vi "FlexMag - 24-03-2023.vi"() -> ()   [LabVIEW 2018] (continued)
                n19188 = flat-sequence {
                  frame #0 {
                    w23535 = sgl 0.5 ("TC2_overspeed_value")
                    n19189 = local read "tension value"() -> (w23537:dbl)
                    n19190 = Wait (ms)(milliseconds to wait=u32 300) -> ()  [unwired: 1 out]
                    n19191 = local write "TC1_set_value"(w23537) -> ()
                    n19192 = local write "TC2_overspeed_value"(w23535) -> ()
                    n19193 = local write "current voltage"(w23535) -> ()
                  }
                  frame #1 {
                    n19194 = local write "TC2_overspeed_set"(TRUE ("TC2 Set moxa")) -> ()
                    n19195 = local write "TC1_auto_set"(TRUE ("TC1_set")) -> ()
                  }
                  frame #2 {
                    n19196 = local write "TC1_overspeed_value"(sgl 0.0 ("TC2_set_value")) -> ()
                    n19197 = local write "TC2_set_value"(sgl 0.0 ("TC2_set_value")) -> ()
                    n19198 = Wait (ms)(milliseconds to wait=u32 300) -> ()  [unwired: 1 out]
                  }
                  frame #3 {
                    n19199 = local write "TC2_auto_set"(TRUE ("TC2_auto_set")) -> ()
                    n19200 = local write "TC1_overspeed_set"(TRUE ("TC2_auto_set")) -> ()
                  }
                }
              }
            }
          }
          frame #10 {
            n19201 = local read "position"() -> (w23545:bool)
            n19202 = case shown="True" w23545 {
              frame False {
              }
              frame True {
                w23547 = TRUE ("CH1_SRV_Direction_Clockwise_DO")
                n19203 = local write "CH1_SRV_Direction_Clockwise_DO"(w23547) -> ()
                n19204 = local write "CH2_SRV_Direction_Clockwise_DO"(w23547) -> ()
                n19205 = local write "CH3_SRV_Direction_Clockwise_DO"(w23547) -> ()
                n19206 = local write "CH4_SRV_Direction_Clockwise_DO"(w23547) -> ()
                n19207 = Wait (ms)(milliseconds to wait=u32 100) -> ()  [unwired: 1 out]
              }
            }
          }
          frame #11 {
            n19208 = local read "position"() -> (w23548:bool)
            n19209 = case shown="True" w23548 {
              frame False {
              }
              frame True {
                n19210 = local write "Tension_Controllers_Start/Stop DO"(TRUE ("CH1_SRV_Direction_Clockwise_DO")) -> ()
                n19211 = Wait (ms)(milliseconds to wait=u32 100) -> ()  [unwired: 1 out]
              }
            }
          }
          frame #12 {
            n19212 = local read "position"() -> (w23552:bool)
            n19213 = case shown="True" w23552 {
              tunnel: w23551 -> [_ w23553]
              frame False {
              }
              frame True {
                n19214 = Wait (ms)(milliseconds to wait=u32 100) -> ()  [unwired: 1 out]
                n19215 = case shown="0, Default" w23553 {
                  frame 0, Default {
                    n19216 = local write "roll error"(TRUE ("roll error")) -> ()
                  }
                  frame 1 {
                    n19217 = local write "CH1_Motor DO"(TRUE ("CH1_Motor DO")) -> ()
                  }
                  frame 2 {
                    n19218 = local write "CH2_Motor DO"(TRUE ("CH1_Motor DO")) -> ()
                  }
                  frame 3 {
                    n19219 = local write "CH3_Motor DO"(TRUE ("CH1_Motor DO")) -> ()
                  }
                  frame 4 {
                    n19220 = local write "CH4_Motor DO"(TRUE ("CH1_Motor DO")) -> ()
                  }
                }
              }
            }
          }
          frame #13 {
            n19221 = stacked-sequence {
              tunnel: w23560 -> [w23561 w23596 _]
              frame #0 {
                n19222 = local read "position"() -> (w23562:bool)
                n19223 = case shown="True" w23562 {
                  tunnel: w23561 -> [_ w23563]
                  frame False {
                  }
                  frame True {
                    n19224 = case shown="4" w23563 {
                      frame 0, Default {
                      }
                      frame 1 {
                        n19225 = while {
                          stop <- w23566 stop-if-true
                          n19226 = local read "Ch1_srv1_counter DI"() -> (w23569:bool)
                          n19227 = Wait Until Next ms Multiple(millisecond multiple=u32 100) -> ()  [unwired: 1 out]
                          n19228 = local read "position"() -> (w23567:bool)
                          n19229 = case shown="True" w23569 {
                            tunnel: [FALSE TRUE] -> w23565
                            frame False {
                            }
                            frame True {
                            }
                          }
                          n19230 = Not(x=w23567) -> (.not. x?=w23564:bool)
                          n19231 = Or(x=w23565, y=w23564) -> (x .or. y?=w23566:bool)
                        }
                      }
                      frame 2 {
                        n19232 = while {
                          stop <- w23574 stop-if-true
                          n19233 = local read "Ch2_srv1_counter DI"() -> (w23577:bool)
                          n19234 = Wait Until Next ms Multiple(millisecond multiple=u32 100) -> ()  [unwired: 1 out]
                          n19235 = local read "position"() -> (w23575:bool)
                          n19236 = case shown="True" w23577 {
                            tunnel: [FALSE TRUE] -> w23573
                            frame False {
                            }
                            frame True {
                            }
                          }
                          n19237 = Not(x=w23575) -> (.not. x?=w23572:bool)
                          n19238 = Or(x=w23573, y=w23572) -> (x .or. y?=w23574:bool)
                        }
                      }
                      frame 3 {
                        n19239 = while {
                          stop <- w23582 stop-if-true
                          n19240 = local read "Ch3_srv1_counter DI"() -> (w23585:bool)
                          n19241 = Wait Until Next ms Multiple(millisecond multiple=u32 100) -> ()  [unwired: 1 out]
                          n19242 = local read "position"() -> (w23583:bool)
                          n19243 = case shown="True" w23585 {
                            tunnel: [FALSE TRUE] -> w23581
                            frame False {
                            }
                            frame True {
                            }
                          }
                          n19244 = Not(x=w23583) -> (.not. x?=w23580:bool)
                          n19245 = Or(x=w23581, y=w23580) -> (x .or. y?=w23582:bool)
                        }
                      }
                      frame 4 {
                        n19246 = while {
                          stop <- w23590 stop-if-true
                          n19247 = local read "Ch4_srv1_counter DI"() -> (w23593:bool)
                          n19248 = Wait Until Next ms Multiple(millisecond multiple=u32 100) -> ()  [unwired: 1 out]
                          n19249 = local read "position"() -> (w23591:bool)
                          n19250 = case shown="True" w23593 {
                            tunnel: [FALSE TRUE] -> w23589
                            frame False {
                            }
                            frame True {
                            }
                          }
                          n19251 = Not(x=w23591) -> (.not. x?=w23588:bool)
                          n19252 = Or(x=w23589, y=w23588) -> (x .or. y?=w23590:bool)
                        }
                      }
                    }
                  }
                }
              }
              frame #1 {
                n19253 = local read "position"() -> (w23597:bool)
                n19254 = case shown="True" w23597 {
                  tunnel: w23596 -> [_ w23598]
                  frame False {
                  }
                  frame True {
                    n19255 = case shown="0, Default" w23598 {
                      frame 0, Default {
                        n19256 = local write "roll error"(TRUE ("roll error")) -> ()
                      }
                      frame 1 {
                        n19257 = while {
                          stop <- w23602 stop-if-true
                          n19258 = local read "Ch1_srv1_counter DI"() -> (w23605:bool)
                          n19259 = Wait Until Next ms Multiple(millisecond multiple=u32 100) -> ()  [unwired: 1 out]
                          n19260 = local read "position"() -> (w23603:bool)
                          n19261 = case shown="False" w23605 {
                            tunnel: [TRUE FALSE] -> w23601
                            frame False {
                              n19262 = local write "CH1_Motor DO"(FALSE ("CH1_Motor DO")) -> ()
                            }
                            frame True {
                            }
                          }
                          n19263 = Not(x=w23603) -> (.not. x?=w23600:bool)
                          n19264 = Or(x=w23601, y=w23600) -> (x .or. y?=w23602:bool)
                        }
                      }
                      frame 2 {
                        n19265 = while {
                          stop <- w23611 stop-if-true
                          n19266 = local read "Ch2_srv1_counter DI"() -> (w23614:bool)
                          n19267 = Wait Until Next ms Multiple(millisecond multiple=u32 100) -> ()  [unwired: 1 out]
                          n19268 = local read "position"() -> (w23612:bool)
                          n19269 = case shown="False" w23614 {
                            tunnel: [TRUE FALSE] -> w23610
                            frame False {
                              n19270 = local write "CH2_Motor DO"(FALSE ("CH1_Motor DO")) -> ()
                            }
                            frame True {
                            }
                          }
                          n19271 = Not(x=w23612) -> (.not. x?=w23609:bool)
                          n19272 = Or(x=w23610, y=w23609) -> (x .or. y?=w23611:bool)
                        }
                      }
                      frame 3 {
                        n19273 = while {
                          stop <- w23620 stop-if-true
                          n19274 = local read "Ch3_srv1_counter DI"() -> (w23623:bool)
                          n19275 = Wait Until Next ms Multiple(millisecond multiple=u32 100) -> ()  [unwired: 1 out]
                          n19276 = local read "position"() -> (w23621:bool)
                          n19277 = case shown="False" w23623 {
                            tunnel: [TRUE FALSE] -> w23619
                            frame False {
                              n19278 = local write "CH3_Motor DO"(FALSE ("CH1_Motor DO")) -> ()
                            }
                            frame True {
                            }
                          }
                          n19279 = Not(x=w23621) -> (.not. x?=w23618:bool)
                          n19280 = Or(x=w23619, y=w23618) -> (x .or. y?=w23620:bool)
                        }
                      }
                      frame 4 {
                        n19281 = while {
                          stop <- w23629 stop-if-true
                          n19282 = local read "Ch4_srv1_counter DI"() -> (w23632:bool)
                          n19283 = Wait Until Next ms Multiple(millisecond multiple=u32 100) -> ()  [unwired: 1 out]
                          n19284 = local read "position"() -> (w23630:bool)
                          n19285 = case shown="False" w23632 {
                            tunnel: [TRUE FALSE] -> w23628
                            frame False {
                              n19286 = local write "CH4_Motor DO"(FALSE ("CH1_Motor DO")) -> ()
                            }
                            frame True {
                            }
                          }
                          n19287 = Not(x=w23630) -> (.not. x?=w23627:bool)
                          n19288 = Or(x=w23628, y=w23627) -> (x .or. y?=w23629:bool)
                        }
                      }
                    }
                  }
                }
              }
              frame #2 {
                w23636 = FALSE ("forward roll")
                n19289 = local write "Tension_Controllers_Start/Stop DO"(w23636) -> ()
                n19290 = local write "CH1_Motor DO"(w23636) -> ()
                n19291 = local write "CH2_Motor DO"(w23636) -> ()
                n19292 = local write "CH3_Motor DO"(w23636) -> ()
                n19293 = local write "CH4_Motor DO"(w23636) -> ()
                n19294 = local write "position"(FALSE ("position")) -> ()
                n19295 = Wait (ms)(milliseconds to wait=u32 300) -> ()  [unwired: 1 out]
              }
            }
          }
        }
      }
    }
  }
  n19296 = while {
    stop <- FALSE stop-if-true
    n19297 = Wait Until Next ms Multiple(millisecond multiple=u32 300) -> ()  [unwired: 1 out]
    n19298 = case shown="True" "calculate" {
      frame False {
      }
      frame True {
        n19299 = stacked-sequence {
          frame #0 {
            w23643 = 0.0 ("lap number right target")
            n19300 = local read "initial right diameter"() -> (w23642:dbl)
            n19301 = local write "final right diameter"(w23642) -> ()
            n19302 = local write "lap number right target"(w23643) -> ()
            n19303 = local write "total interval"(w23643) -> ()
          }
          frame #1 {
            n19304 = while {
              stop <- w23654 stop-if-true
              n19305 = local read "web thickness"() -> (w23651:dbl)
              n19306 = local read "final right diameter"() -> (w23645:dbl)
              n19307 = local read "lap number right target"() -> (w23659:dbl)
              n19308 = local read "total interval"() -> (w23648:dbl)
              n19309 = Multiply(x=w23651, y=0.002) -> (x*y=w23652:dbl)
              n19310 = Multiply(x=w23645, y=0.1) -> (x*y=w23646:dbl)
              n19311 = local read "target interval"() -> (w23655:dbl)
              n19312 = Add(x=w23645, y=w23652) -> (x+y=w23653:dbl)
              n19313 = Multiply(x=3.141592653589793, y=w23646) -> (x*y=w23649:dbl)
              n19314 = Add(x=w23659, y=1.0) -> (x+y=w23660:dbl)
              n19315 = local write "lap number right target"(w23660) -> ()
              n19316 = local write "final right diameter"(w23653) -> ()
              n19317 = Add(x=w23648, y=w23649) -> (x+y=w23647:dbl)
              n19318 = Greater Or Equal?(x=w23647, y=w23655) -> (x >= y?=w23654:bool)
              n19319 = local write "total interval"(w23647) -> ()
              n19320 = Wait Until Next ms Multiple(millisecond multiple=u32 50) -> ()  [unwired: 1 out]
            }
          }
          frame #2 {
            n19321 = local read "initial right diameter"() -> (w23673:dbl)
            n19322 = local read "final right diameter"() -> (w23661:dbl)
            n19323 = local read "web speed"() -> (w23670:dbl)
            n19324 = local read "web speed"() -> (w23662:dbl)
            n19325 = Multiply(x=w23673, y=3.141592653589793) -> (x*y=w23671:dbl)
            n19326 = Multiply(x=w23661, y=3.141592653589793) -> (x*y=w23674:dbl)
            n19327 = Divide(x=w23670, y=w23671) -> (x/y=w23667:dbl)
            n19328 = Divide(x=w23662, y=w23674) -> (x/y=w23669:dbl)
            n19329 = Multiply(x=w23669, y=10.0) -> (x*y=→"min circular speed":dbl)
            n19330 = Multiply(x=w23667, y=10.0) -> (x*y=→"max circular speed":dbl)
            n19331 = Wait (ms)(milliseconds to wait=u32 100) -> ()  [unwired: 1 out]
          }
          frame #3 {
            # "1/50 redüktör"
            # "1000rpm 10volts"
            n19332 = local read "min circular speed"() -> (w23681:dbl)
            n19333 = local read "max circular speed"() -> (w23685:dbl)
            n19334 = Multiply(x=0.01, y=50.0 ("x")) -> (x*y=w23682:dbl)
            n19335 = Multiply(x=w23685, y=w23682) -> (x*y=w23676:dbl)
            n19336 = Multiply(x=w23682, y=w23681) -> (x*y=w23677:dbl)
            n19337 = local write "final output voltage"(w23677) -> ()
            n19338 = local read "lap number right target"() -> (w23679:dbl)
            n19339 = Subtract(x=w23676, y=w23677) -> (x-y=w23680:dbl)
            n19340 = local write "initial output voltage"(w23676) -> ()
            n19341 = Divide(x=w23680, y=w23679) -> (x/y=w23678:dbl)
            n19342 = local write "decreasing voltage"(w23678) -> ()
          }
          frame #4 {
            n19343 = local write "calculate"(FALSE ("calculate")) -> ()
          }
        }
      }
    }
  }
  n19344 = while {
    stop <- FALSE stop-if-true
    n19345 = Wait Until Next ms Multiple(millisecond multiple=u32 300) -> ()  [unwired: 1 out]
    n19346 = case shown="True" "tension check active" {
      frame False {
      }
      frame True {
        n19347 = local read "Tension_Controllers_Start/Stop DO"() -> (w23718:bool)
        n19348 = local read "CH1_Motor DO"() -> (w23723:bool)
        n19349 = local read "CH2_Motor DO"() -> (w23722:bool)
        n19350 = local read "CH3_Motor DO"() -> (w23721:bool)
        n19351 = local read "CH4_Motor DO"() -> (w23720:bool)
        n19352 = Compound Arithmetic op=OR(w23723, w23722, w23721, w23720) -> (w23717:bool)
        n19353 = And(x=w23718, y=w23717) -> (x .and. y?=w23719:bool)
        n19354 = feedback #338() -> (w23715:bool)  [unwired: 1 in]
        n19355 = case shown="True" w23719 {
          tunnel: [TRUE ("Dc_auto_off") w23729] -> w23716
          tunnel: w23715 -> [_ w23728]
          tunnel: "check both tensions" -> [_ w23727]
          frame False {
          }
          frame True {
            n19356 = case shown="True" w23727 {
              tunnel: "tension check value" -> [w23731 w23739]
              tunnel: [w23730 w23736] -> w23725
              frame False {
                n19357 = local read "forward roll"() -> (w23733:bool)
                n19358 = case shown="False" w23733 {
                  tunnel: [w23734 w23735] -> w23732
                  frame False {
                    n19359 = local read "TC2_measure_value"() -> (w23734:sgl)
                  }
                  frame True {
                    n19360 = local read "TC1_measure_value"() -> (w23735:sgl)
                  }
                }
                n19361 = Greater Or Equal?(x=w23732, y=w23731) -> (x >= y?=w23730:bool)
              }
              frame True {
                n19362 = local read "TC1_measure_value"() -> (w23741:sgl)
                n19363 = local read "TC2_measure_value"() -> (w23740:sgl)
                n19364 = Greater Or Equal?(x=w23741, y=w23739) -> (x >= y?=w23738:bool)
                n19365 = Greater Or Equal?(x=w23740, y=w23739) -> (x >= y?=w23737:bool)
                n19366 = Or(x=w23738, y=w23737) -> (x .or. y?=w23736:bool)
              }
            }
            n19367 = case shown="True" w23725 {
              tunnel: [TRUE ("Dc_auto_off") FALSE] -> w23729
              tunnel: w23728 -> [_ w23743]
              frame False {
              }
              frame True {
                n19368 = call "Elapsed Time191"("Reset"=w23743) -> ("Elapsed Time (s)"=w23746:dbl)  [unwired: 11 in, 7 out]
                n19369 = Greater?(x=w23746, y="tension check (sec)") -> (0:w23744:bool)
                n19370 = case shown="True" w23744 {
                  frame False {
                  }
                  frame True {
                    n19371 = local write "Warning Message"("Rolling Problem !\nToo much Tension !" ("Warning Message")) -> ()
                    n19372 = local write "roll error"(TRUE ("roll error")) -> ()
                  }
                }
              }
            }
          }
        }
        n19373 = feedback-in #338(w23716) -> ()
      }
    }
    n19374 = case shown="True" "speed check active" {
      frame False {
      }
      frame True {
        n19375 = local read "Tension_Controllers_Start/Stop DO"() -> (w23698:bool)
        n19376 = local read "CH1_Motor DO"() -> (w23694:bool)
        n19377 = local read "CH2_Motor DO"() -> (w23695:bool)
        n19378 = local read "CH3_Motor DO"() -> (w23696:bool)
        n19379 = local read "CH4_Motor DO"() -> (w23697:bool)
        n19380 = Compound Arithmetic op=OR(w23694, w23695, w23696, w23697) -> (w23699:bool)
        n19381 = feedback #339() -> (w23691:bool)  [unwired: 1 in]
        n19382 = And(x=w23698, y=w23699) -> (x .and. y?=w23693:bool)
        n19383 = case shown="True" w23693 {
          tunnel: [TRUE ("Dc_auto_off") w23702] -> w23692
          tunnel: w23691 -> [_ w23701]
          frame False {
          }
          frame True {
            n19384 = local read "process variable"() -> (w23705:dbl)
            n19385 = Less Or Equal?(x=w23705, y="speed compare value") -> (x <= y?=w23703:bool)
            n19386 = case shown="True" w23703 {
              tunnel: [TRUE ("Dc_auto_off") FALSE] -> w23702
              tunnel: w23701 -> [_ w23710]
              frame False {
              }
              frame True {
                n19387 = call "Elapsed Time193"("Reset"=w23710) -> ("Elapsed Time (s)"=w23709:dbl)  [unwired: 11 in, 7 out]
                n19388 = Greater?(x=w23709, y="speed check (sec)") -> (0:w23707:bool)
                n19389 = case shown="True" w23707 {
                  frame False {
                  }
                  frame True {
                    n19390 = local write "roll error"(TRUE ("roll error")) -> ()
                    n19391 = local write "Warning Message"("Rolling Problem !\nNo Speed !" ("Warning Message")) -> ()
                  }
                }
              }
            }
          }
        }
        n19392 = feedback-in #339(w23692) -> ()
      }
    }
  }
  n19393 = while {
    stop <- FALSE stop-if-true
    n19394 = flat-sequence {
      frame #0 {
        n19395 = local read "keysight readout"() -> (w23760:dbl)
        n19396 = In Range and Coerce(upper limit="output limit max", x=w23760, lower limit="output limit min") -> (coerced(x)=w23754:dbl)  [unwired: 1 out]
        "freq readout" <- w23754
        n19397 = Divide(x="speed coef", y="freq coef") -> (x/y=w23755:sgl)
        n19398 = Multiply(x=w23754, y=w23755) -> (x*y=→"process variable":dbl)
      }
      frame #1 {
        n19399 = local read "process variable"() -> (w23761:dbl)
        n19400 = call-poly <vilib>:"PID.vi"("output range"="output range", "dt (s)"="dt (s)", "PID gains"="PID gains", "process variable"=w23761, "setpoint"="setpoint") -> ("output"=→"output_pid" →"Waveform Chart":dbl)  [unwired: 5 in, 1 out]
      }
    }
    n19401 = Wait Until Next ms Multiple(millisecond multiple=u32 300) -> ()  [unwired: 1 out]
    n19402 = property on="pid graph" class="TabCtl (strict)"("Visible"="show graph") -> ()  [unwired: 2 in, 2 out]
  }
  n19403 = disable-structure shown="Disabled" {
    frame Disabled {
      n19404 = while {
        stop <- FALSE stop-if-true
        n19405 = Wait Until Next ms Multiple(millisecond multiple=u32 300) -> ()  [unwired: 1 out]
        n19406 = case shown="True" "pid output" {
          frame False {
          }
          frame True {
            n19407 = stacked-sequence {
              frame #0 {
                n19408 = while {
                  i -> [w23776]
                  stop <- w23771 stop-if-true
                  n19409 = local read "final output voltage"() -> (w23773:dbl)
                  n19410 = Wait Until Next ms Multiple(millisecond multiple=u32 300) -> ()  [unwired: 1 out]
                  n19411 = Multiply(x=w23776, y=0.5 ("lower limit")) -> (x*y=w23774:dbl)
                  n19412 = Greater Or Equal?(x=w23774, y=w23773) -> (x >= y?=w23772:bool)
                  n19413 = In Range and Coerce(upper limit=w23773, x=w23774, lower limit=0.5) -> (coerced(x)=w23770:dbl)  [unwired: 1 out]
                  n19414 = case shown="True" w23772 {
                    tunnel: [FALSE ("pid output") TRUE ("pid output")] -> w23771
                    frame False {
                    }
                    frame True {
                      n19415 = local write "pid output"(FALSE ("pid output")) -> ()
                    }
                  }
                  n19416 = Bundle("final output voltage"=w23770, "final output voltage"=w23770) -> (w23779:T17)  [unwired: 1 in]
                  n19417 = local write "output range"(w23779) -> ()
                }
              }
              frame #1 {
                n19418 = local read "initial output voltage"() -> (w23785:dbl)
                n19419 = local read "final output voltage"() -> (w23784:dbl)
                n19420 = Wait (ms)(milliseconds to wait=u32 100) -> ()  [unwired: 1 out]
                n19421 = Bundle("initial output voltage"=w23785, "final output voltage"=w23784) -> (w23786:T18)  [unwired: 1 in]
                n19422 = local write "output range"(w23786) -> ()
              }
            }
          }
        }
      }
    }
    frame Enabled {
    }
  }
  n19423 = local write "dep. for?"(w1) -> ()
  n19424 = while {
    stop <- FALSE stop-if-true
    n19425 = local read "process file list"() -> (w23790:string)
    n19426 = Wait Until Next ms Multiple(millisecond multiple=u32 300) -> ()  [unwired: 1 out]
    n19427 = Match Pattern(string=w23790, regular expression="\r\n") -> (before substring=w23791:string)  [unwired: 1 in, 3 out]
    n19428 = Equal?(x=w23791, y="FlexMag Process File") -> (x = y?=w23787:bool)
    n19429 = case shown="True" "coating start" {
      tunnel: w23787 -> [_ w23796]
      frame False {
      }
      frame True {
        n19430 = case shown="True" w23796 {
          frame False {
            n19431 = flat-sequence {
              frame #0 {
                n19432 = local write "Buzzer DO"(TRUE ("Buzzer DO")) -> ()
                n19433 = local write "coating start"(FALSE ("coating start")) -> ()
                n19434 = local write "Warning Message"("Please Enter a proper Process File !" ("Warning Message")) -> ()
              }
              frame #1 {
                n19435 = Wait (ms)(milliseconds to wait=u32 3000) -> ()  [unwired: 1 out]
              }
              frame #2 {
                n19436 = local write "Buzzer DO"(FALSE ("Buzzer DO")) -> ()
              }
            }
          }
          frame True {
            n19437 = while {
              i -> [w23809]
              stop <- "coating process done" stop-if-true
              n19438 = Increment(x=w23809) -> (x+1=w23804:i32)
              n19439 = local read "process file list"() -> (w23817:string)
              n19440 = Number To Decimal String(number=w23804) -> (decimal integer string=w23816:string)  [unwired: 1 in]
              n19441 = Concatenate Strings(w23816, "-)") -> (w23814:string)
              n19442 = Wait Until Next ms Multiple(millisecond multiple=u32 300) -> ()  [unwired: 1 out]
              n19443 = Increment(x=w23804) -> (x+1=w23807:i32)
              n19444 = Match Pattern(string=w23817, regular expression=w23814) -> (after substring=w23813:string)  [unwired: 1 in, 3 out]
              n19445 = Number To Decimal String(number=w23807) -> (decimal integer string=w23806:string)  [unwired: 1 in]
              n19446 = Concatenate Strings(w23806, "-)") -> (w23803:string)
              n19447 = Match Pattern(string=w23813, regular expression=w23803) -> (before substring=w23808:string)  [unwired: 1 in, 3 out]
              n19448 = Equal?(x="", y=w23808) -> (x = y?=w23811:bool)
              n19449 = case shown="False" w23811 {
                tunnel: w23808 -> [w23819 _]
                tunnel: w23804 -> [w23818 _]
                frame False {
                  # "process available"
                  n19450 = stacked-sequence {
                    tunnel: w23819 -> [w23825 _]
                    tunnel: w23818 -> [w23821 _]
                    frame #0 {
                      n19451 = local read "coating start"() -> (w23820:bool)
                      n19452 = case shown="False" w23820 {
                        tunnel: [w23828 w23829] -> w23822
                        tunnel: w23821 -> [_ w23829]
                        frame False {
                          n19453 = local read "current recipe number"() -> (w23828:i32)
                        }
                        frame True {
                        }
                      }
                      "current recipe number" <- w23822
                      n19454 = local read "cassette position selection"() -> (w23823:u16)
                      n19455 = Match Pattern(string=w23825, regular expression="\r\n") -> (before substring=w23826:string)  [unwired: 1 in, 3 out]
                      "process file list 2" <- w23826
                      n19456 = case shown="0, Default" w23823 {
                        frame 0, Default {
                          n19457 = local write "coating error"(TRUE ("coating error")) -> ()
                          n19458 = local write "Warning Message"("Choose Cassette Position !" ("Warning Message")) -> ()
                        }
                        frame 1 {
                        }
                        frame 2 {
                        }
                        frame 3 {
                        }
                        frame 4 {
                        }
                      }
                      n19459 = stacked-sequence {
                        tunnel: w23826 -> [w23834 _ _ _ _]
                        frame #0 {
                          n19460 = String To Path(string=w23834) -> (path=→"path for loading recipe":path)
                          n19461 = Wait (ms)(milliseconds to wait=u32 500) -> ()  [unwired: 1 out]
                        }
                        frame #1 {
                          n19462 = Wait (ms)(milliseconds to wait=u32 1000) -> ()  [unwired: 1 out]
                        }
                        frame #2 {
                          n19463 = local write "load recipe from path"(TRUE ("load recipe from path")) -> ()
                        }
                        frame #3 {
                          n19464 = Wait (ms)(milliseconds to wait=u32 1000) -> ()  [unwired: 1 out]
                        }
                        frame #4 {
                          n19465 = while {
                            i -> [w23840]
                            stop <- w23844 stop-if-true
                            n19466 = local read "load recipe from path"() -> (w23841:bool)
                            n19467 = local read "ABORT"() -> (w23843:bool)
                            n19468 = Wait Until Next ms Multiple(millisecond multiple=u32 1000) -> ()  [unwired: 1 out]
                            n19469 = Greater?(x=w23840, y=u32 30 ("millisecond multiple")) -> (0:w23838:bool)
                            n19470 = Not(x=w23841) -> (.not. x?=w23842:bool)
                            n19471 = Compound Arithmetic op=OR(w23842, w23843, w23838) -> (w23844:bool)
                            n19472 = local write "coating error"(w23838) -> ()
                          }
                        }
                      }
                      n19473 = local write "System Status"("COATING MODE ACTIVE" ("System Status")) -> ()
                    }
                    frame #1 {
                      n19474 = local read "R Recipe Selection"() -> (w23846:u16)
                      n19475 = case shown="0, Default" w23846 {
                        frame 0, Default {
                          # "SINGLE PROCESS"
                          n19476 = local read "R single process selection"() -> (w23847:enum32{"microwave", "dcsputter", "rfsputter"})
                          n19477 = case shown="\"dcsputter\"" w23847 {
                            frame "microwave", Default {
                            }
                            frame "dcsputter" {
                              # "DC SPUTTER"
                              n19478 = local read "R DC Sputter Chamber Selection"() -> (w23848:enum32{"chamber II", "chamber III"})
                              n19479 = case shown="\"chamber III\"" w23848 {
                                frame "chamber II", Default {
                                # "CH II"
                                n19480 = disable-structure shown="Enabled" {
                                disable-tunnel: [w23850 TRUE] -> w23849
                                frame Disabled {
                                n19481 = local read "ch2 ch pg torr"() -> (w23852:dbl)
                                n19482 = local read "ch2 cc torr"() -> (w23851:dbl)
                                n19483 = Less Or Equal?(x=w23852, y=0.005) -> (x <= y?=w23855:bool)
                                n19484 = Less Or Equal?(x=w23851, y=0.005) -> (x <= y?=w23856:bool)
                                n19485 = And(x=w23855, y=w23856) -> (x .and. y?=w23850:bool)
                                }
                                frame Enabled {
                                }
                                }
                                n19486 = case shown="True" w23849 {
                                frame False {
                                n19487 = local write "coating error"(TRUE ("coating error")) -> ()
                                n19488 = local write "Warning Message"("Automatic Coating Process is canceled !\nCH2 Pressure should be under 5E-3 Torr .." ("Warning Message")) -> ()
                                }
                                frame True {
                                n19489 = stacked-sequence {
                                frame #0 {
                                }
                                frame #1 {
                                n19490 = stacked-sequence {
                                frame #0 {
                                n19491 = local read "abort ch2"() -> (w23860:bool)
                                n19492 = case shown="False" w23860 {
                                frame False {
                                n19493 = local read "coating start"() -> (w23861:bool)
                                n19494 = case shown="True" w23861 {
                                frame False {
                                }
                                frame True {
                                n19495 = local read "casette_ch2_gui"() -> (w23863:bool)
                                n19496 = Wait (ms)(milliseconds to wait=u32 100) -> ()  [unwired: 1 out]
                                n19497 = case shown="False" w23863 {
                                frame False {
                                n19498 = stacked-sequence {
                                frame #0 {
                                n19499 = flat-sequence {
                                frame #0 {
                                n19500 = local write "target chamber"(2.0 ("target chamber")) -> ()
                                n19501 = Wait (ms)(milliseconds to wait=u32 100) -> ()  [unwired: 1 out]
                                }
                                frame #1 {
                                n19502 = Wait (ms)(milliseconds to wait=u32 1000) -> ()  [unwired: 1 out]
                                }
                                frame #2 {
                                n19503 = local write "transfer vacuum auto"(TRUE ("transfer vacuum")) -> ()
                                }
                                }
                                }
                                frame #1 {
                                n19504 = while {
                                i -> [w23871]
                                stop <- w23873 stop-if-true
                                # "20min"
                                n19505 = local read "present location"() -> (w23877:dbl)
                                n19506 = local read "casette_ch2_gui"() -> (w23869:bool)
                                n19507 = local read "abort ch2"() -> (w23872:bool)
                                n19508 = Equal?(x=w23877, y=2.0) -> (x = y?=w23875:bool)
                                n19509 = Greater?(x=w23871, y=1200) -> (0:w23868:bool)
                                n19510 = local write "trns error"(w23868) -> ()
                                n19511 = Compound Arithmetic op=OR(w23872, w23875, w23869, w23868) -> (w23873:bool)
                                n19512 = Wait Until Next ms Multiple(millisecond multiple=u32 1000) -> ()  [unwired: 1 out]
                                }
                                }
                                }
                                }
                                frame True {
                                }
                                }
                                }
                                }
                                }
                                frame True {
                                }
                                }
                                }
                                frame #1 {
                                n19513 = local read "abort ch2"() -> (w23878:bool)
                                n19514 = case shown="False" w23878 {
                                frame False {
                                n19515 = local read "coating start"() -> (w23879:bool)
                                n19516 = case shown="True" w23879 {
                                frame False {
                                }
                                frame True {
                                n19517 = Wait (ms)(milliseconds to wait=u32 100) -> ()  [unwired: 1 out]
                                n19518 = local write "System Status"("COATING MODE ACTIVE" ("System Status")) -> ()
                                "coating ch2 led 1" <- TRUE ("coating ch2 led 1")
                                }
                                }
                                }
                                frame True {
                                }
                                }
                                }
                                }
                                }
                                frame #2 {
                                # "water"
                                n19519 = stacked-sequence {
                                frame #0 {
                                # "ch1 water off"
                                n19520 = local read "abort ch2"() -> (w23883:bool)
                                n19521 = case shown="False" w23883 {
                                frame False {
                                n19522 = local read "coating start"() -> (w23884:bool)
                                n19523 = case shown="True" w23884 {
                                frame False {
                                }
                                frame True {
                                n19524 = while {
                                i -> [w23887]
                                stop <- w23889 stop-if-true
                                n19525 = Greater Or Equal?(x=w23887, y=100) -> (x >= y?=w23888:bool)
                                n19526 = case shown="True" w23888 {
                                frame False {
                                }
                                frame True {
                                n19527 = local write "coating error"(TRUE ("coating error")) -> ()
                                n19528 = local write "Warning Message"("Automatic Coating Process is canceled !\nCH1 Water Flow Problem.." ("Warning Message")) -> ()
                                }
                                }
                                n19529 = local read "CH1_WFC_DI"() -> (w23893:bool)
                                n19530 = case shown="True" w23893 {
                                tunnel: [TRUE ("CH2_WFC_DO") FALSE ("CH2_WFC_DO")] -> w23892
                                frame False {
                                }
                                frame True {
                                n19531 = Wait Until Next ms Multiple(millisecond multiple=u32 200) -> ()  [unwired: 1 out]
                                n19532 = local write "CH1_WFC_DO"(FALSE ("CH2_WFC_DO")) -> ()
                                }
                                }
                                n19533 = local read "coating start"() -> (w23891:bool)
                                n19534 = local read "abort ch2"() -> (w23885:bool)
                                n19535 = Not(x=w23891) -> (.not. x?=w23890:bool)
                                n19536 = Compound Arithmetic op=OR(w23892, w23890, w23885) -> (w23889:bool)
                                }
                                }
                                }
                                }
                                frame True {
                                }
                                }
                                }
                                frame #1 {
                                # "ch3 water off"
                                n19537 = local read "abort ch2"() -> (w23900:bool)
                                n19538 = case shown="False" w23900 {
                                frame False {
                                n19539 = local read "coating start"() -> (w23901:bool)
                                n19540 = case shown="True" w23901 {
                                frame False {
                                }
                                frame True {
                                n19541 = while {
                                i -> [w23904]
                                stop <- w23906 stop-if-true
                                n19542 = Greater Or Equal?(x=w23904, y=100) -> (x >= y?=w23905:bool)
                                n19543 = case shown="True" w23905 {
                                frame False {
                                }
                                frame True {
                                n19544 = local write "coating error"(TRUE ("coating error")) -> ()
                                n19545 = local write "Warning Message"("Automatic Coating Process is canceled !\nCH3 Water Flow Problem.." ("Warning Message")) -> ()
                                }
                                }
                                n19546 = local read "CH3_WFC_DI"() -> (w23910:bool)
                                n19547 = case shown="True" w23910 {
                                tunnel: [TRUE ("CH2_WFC_DO") FALSE ("CH2_WFC_DO")] -> w23909
                                frame False {
                                }
                                frame True {
                                n19548 = Wait Until Next ms Multiple(millisecond multiple=u32 200) -> ()  [unwired: 1 out]
                                n19549 = local write "CH3_WFC_DO"(FALSE ("CH2_WFC_DO")) -> ()
                                }
                                }
                                n19550 = local read "coating start"() -> (w23908:bool)
                                n19551 = local read "abort ch2"() -> (w23902:bool)
                                n19552 = Not(x=w23908) -> (.not. x?=w23907:bool)
                                n19553 = Compound Arithmetic op=OR(w23909, w23907, w23902) -> (w23906:bool)
                                }
                                }
                                }
                                }
                                frame True {
                                }
                                }
                                }
                                frame #2 {
                                # "ch4 water off"
                                n19554 = local read "abort ch2"() -> (w23917:bool)
                                n19555 = case shown="False" w23917 {
                                frame False {
                                n19556 = local read "coating start"() -> (w23918:bool)
                                n19557 = case shown="True" w23918 {
                                frame False {
                                }
                                frame True {
                                n19558 = while {
                                i -> [w23921]
                                stop <- w23923 stop-if-true
                                n19559 = Greater Or Equal?(x=w23921, y=100) -> (x >= y?=w23922:bool)
                                n19560 = case shown="True" w23922 {
                                frame False {
                                }
                                frame True {
                                n19561 = local write "coating error"(TRUE ("coating error")) -> ()
                                n19562 = local write "Warning Message"("Automatic Coating Process is canceled !\nCH4 Water Flow Problem.." ("Warning Message")) -> ()
                                }
                                }
                                n19563 = local read "CH4_WFC_DI"() -> (w23927:bool)
                                n19564 = case shown="True" w23927 {
                                tunnel: [TRUE ("CH2_WFC_DO") FALSE ("CH2_WFC_DO")] -> w23926
                                frame False {
                                }
                                frame True {
                                n19565 = Wait Until Next ms Multiple(millisecond multiple=u32 200) -> ()  [unwired: 1 out]
                                n19566 = local write "CH4_WFC_DO"(FALSE ("CH2_WFC_DO")) -> ()
                                }
                                }
                                n19567 = local read "coating start"() -> (w23925:bool)
                                n19568 = local read "abort ch2"() -> (w23919:bool)
                                n19569 = Not(x=w23925) -> (.not. x?=w23924:bool)
                                n19570 = Compound Arithmetic op=OR(w23926, w23924, w23919) -> (w23923:bool)
                                }
                                }
                                }
                                }
                                frame True {
                                }
                                }
                                }
                                frame #3 {
                                # "ch2 water on"
                                n19571 = local read "abort ch2"() -> (w23934:bool)
                                n19572 = case shown="False" w23934 {
                                frame False {
                                n19573 = local read "coating start"() -> (w23935:bool)
                                n19574 = case shown="True" w23935 {
                                frame False {
                                }
                                frame True {
                                n19575 = while {
                                i -> [w23938]
                                stop <- w23940 stop-if-true
                                n19576 = Greater Or Equal?(x=w23938, y=100) -> (x >= y?=w23939:bool)
                                n19577 = case shown="True" w23939 {
                                frame False {
                                }
                                frame True {
                                n19578 = local write "coating error"(TRUE ("coating error")) -> ()
                                n19579 = local write "Warning Message"("Automatic Coating Process is canceled !\nCH2 Water Flow Problem.." ("Warning Message")) -> ()
                                }
                                }
                                n19580 = local read "CH2_WFC_DI"() -> (w23944:bool)
                                n19581 = case shown="False" w23944 {
                                tunnel: [FALSE ("CH2_WFC_DO") TRUE ("CH2_WFC_DO")] -> w23943
                                frame False {
                                n19582 = Wait Until Next ms Multiple(millisecond multiple=u32 200) -> ()  [unwired: 1 out]
                                n19583 = local write "CH2_WFC_DO"(TRUE ("CH2_WFC_DO")) -> ()
                                }
                                frame True {
                                }
                                }
                                n19584 = local read "coating start"() -> (w23942:bool)
                                n19585 = local read "abort ch2"() -> (w23936:bool)
                                n19586 = Not(x=w23942) -> (.not. x?=w23941:bool)
                                n19587 = Compound Arithmetic op=OR(w23943, w23941, w23936) -> (w23940:bool)
                                }
                                }
                                }
                                }
                                frame True {
                                }
                                }
                                }
                                frame #4 {
                                n19588 = local read "abort ch2"() -> (w23951:bool)
                                n19589 = case shown="False" w23951 {
                                frame False {
                                n19590 = local read "coating start"() -> (w23952:bool)
                                n19591 = case shown="True" w23952 {
                                frame False {
                                }
                                frame True {
                                n19592 = Wait (ms)(milliseconds to wait=u32 100) -> ()  [unwired: 1 out]
                                "coating ch2 led 2" <- TRUE ("coating ch2 led 1")
                                }
                                }
                                }
                                frame True {
                                }
                                }
                                }
                                }
                                }
                                frame #3 {
                                # "ch2 pcgv on"
                                n19593 = stacked-sequence {
                                frame #0 {
                                n19594 = local read "abort ch2"() -> (w23955:bool)
                                n19595 = case shown="False" w23955 {
                                frame False {
                                n19596 = local read "coating start"() -> (w23956:bool)
                                n19597 = case shown="True" w23956 {
                                frame False {
                                }
                                frame True {
                                n19598 = local read "ch2_pcgv_gui"() -> (w23957:bool)
                                n19599 = case shown="False" w23957 {
                                frame False {
                                n19600 = flat-sequence {
                                frame #0 {
                                n19601 = local write "pcgv2 auto open"(TRUE ("pcgv2 auto open")) -> ()
                                }
                                frame #1 {
                                n19602 = Wait (ms)(milliseconds to wait=u32 1000) -> ()  [unwired: 1 out]
                                }
                                frame #2 {
                                n19603 = local write "pcgv2 auto open"(TRUE ("pcgv2 auto open")) -> ()
                                }
                                }
                                }
                                frame True {
                                }
                                }
                                }
                                }
                                }
                                frame True {
                                }
                                }
                                }
                                frame #1 {
                                n19604 = local read "abort ch2"() -> (w23961:bool)
                                n19605 = case shown="False" w23961 {
                                frame False {
                                n19606 = local read "coating start"() -> (w23962:bool)
                                n19607 = case shown="True" w23962 {
                                frame False {
                                }
                                frame True {
                                n19608 = while {
                                i -> [w23965]
                                stop <- w23967 stop-if-true
                                n19609 = Greater Or Equal?(x=w23965, y=100) -> (x >= y?=w23966:bool)
                                n19610 = case shown="True" w23966 {
                                frame False {
                                }
                                frame True {
                                n19611 = local write "coating error"(TRUE ("coating error")) -> ()
                                n19612 = local write "Warning Message"("Automatic Coating Process is canceled !\nCH2 PCGV couldn't be opened.." ("Warning Message")) -> ()
                                }
                                }
                                n19613 = local read "ch2_pcgv_gui"() -> (w23971:bool)
                                n19614 = case shown="True" w23971 {
                                tunnel: [FALSE ("CH2_WFC_DO") TRUE ("CH2_WFC_DO")] -> w23970
                                frame False {
                                n19615 = Wait Until Next ms Multiple(millisecond multiple=u32 200) -> ()  [unwired: 1 out]
                                }
                                frame True {
                                }
                                }
                                n19616 = local read "coating start"() -> (w23969:bool)
                                n19617 = local read "abort ch2"() -> (w23963:bool)
                                n19618 = Not(x=w23969) -> (.not. x?=w23968:bool)
                                n19619 = Compound Arithmetic op=OR(w23970, w23968, w23963) -> (w23967:bool)
                                }
                                }
                                }
                                }
                                frame True {
                                }
                                }
                                }
                                frame #2 {
                                n19620 = local read "abort ch2"() -> (w23977:bool)
                                n19621 = case shown="False" w23977 {
                                frame False {
                                n19622 = local read "coating start"() -> (w23978:bool)
                                n19623 = case shown="True" w23978 {
                                frame False {
                                }
                                frame True {
                                n19624 = Wait (ms)(milliseconds to wait=u32 100) -> ()  [unwired: 1 out]
                                "coating ch2 led 3" <- TRUE ("coating ch2 led 1")
                                }
                                }
                                }
                                frame True {
                                }
                                }
                                }
                                }
                                }
                                frame #4 {
                                # "DC host - communication check"
                                n19625 = stacked-sequence {
                                frame #0 {
                                n19626 = local read "abort ch2"() -> (w23981:bool)
                                n19627 = case shown="False" w23981 {
                                frame False {
                                n19628 = local read "coating start"() -> (w23982:bool)
                                n19629 = case shown="True" w23982 {
                                frame False {
                                }
                                frame True {
                                n19630 = flat-sequence {
                                frame #0 {
                                n19631 = local write "Dc_host_auto"(TRUE ("pcgv2 auto open")) -> ()
                                }
                                frame #1 {
                                n19632 = Wait (ms)(milliseconds to wait=u32 1000) -> ()  [unwired: 1 out]
                                }
                                frame #2 {
                                n19633 = local write "Dc_host_auto"(TRUE ("pcgv2 auto open")) -> ()
                                }
                                }
                                }
                                }
                                }
                                frame True {
                                }
                                }
                                }
                                frame #1 {
                                n19634 = local read "abort ch2"() -> (w23986:bool)